vi "Controle_Manip_Main_GUI_WorkingBackup_211222.vi"() -> ()   [LabVIEW 2019] (continued)
                                }
                                frame #2 {
                                n1244 = local read "Spectrum End Wavelength (nm)"() -> (w1602:dbl)
                                n1245 = local read "Spectrum Step Wavelength (nm)"() -> (w1600:dbl)
                                n1246 = local read "Spectrum Start Wavelength (nm)"() -> (w1599:dbl)
                                n1247 = Subtract(x=w1602, y=w1599) -> (x-y=w1604:dbl)
                                n1248 = Divide(x=w1604, y=w1600) -> (x/y=w1603:dbl)
                                n1249 = Increment(x=w1603) -> (x+1=w1601:dbl)
                                n1250 = for {
                                N: w1601 -> [_]
                                tunnel: w1600 -> [w1607]
                                tunnel: w1599 -> [w1608]
                                shift-right: [w1609] -> w1595
                                shift-left: dbl[] [] -> [w1611]
                                shift-right: [w1612] -> w1596
                                shift-left: dbl[] [] -> [w1613]
                                i -> [w1617]
                                stop <- w1605 stop-if-true
                                n1251 = Multiply(x=w1617, y=w1607) -> (x*y=w1616:dbl)
                                n1252 = Add(x=w1608, y=w1616) -> (x+y=w1606:dbl)
                                n1253 = local read "ESP300 COM Port"() -> (w1615:refnum<visa-resource-name>)
                                n1254 = stacked-sequence {
                                tunnel: w1606 -> [w1620 _ w1627 _]
                                tunnel: w1615 -> [w1625 _ _ _]
                                tunnel: [_ _ w1634 _] -> w1614
                                tunnel: w1613 -> [w1623 _ _ _]
                                tunnel: [w1622 _ _ _] -> w1612
                                tunnel: [_ _ _ w1652] -> w1605
                                frame #0 {
                                w1618 = u16 1 items=["Detection"=1, "Excitation"=2] ("HR mode")
                                n1255 = call "MotorWL2Pos.vi"("Mono2 Center WL"=w1620, "HR mode"=w1618) -> ("Mono2 Position"=w1621:dbl)
                                n1256 = control-ref of="Mono2 Wavelength (nm)"() -> (w1619:refnum<vi>)
                                n1257 = control-ref of="Mono2 Motor Pos"() -> (w1624:refnum<vi>)
                                n1258 = call "subVI_Mono2Go2Posv2.vi"("Mono2 Motor Pos"=w1624, "Mono2 Wavelength (nm)"=w1619, "HR mode"=w1618, "Postion (Unit)"=w1621, "ESP300 COM Port"=w1625) -> ()  [unwired: 2 out]
                                n1259 = Insert Into Array(array=w1623, new element=w1620) -> (w1622:dbl[])  [unwired: 1 in]
                                }
                                frame #1 {
                                n1260 = Wait (ms)(milliseconds to wait=u32 20) -> ()  [unwired: 1 out]
                                }
                                frame #2 {
                                n1261 = local read "Photodiode error out"() -> (w1628:errorcluster)
                                n1262 = local read "Photodiode handle out"() -> (w1631:refnum<visa-resource-name>)
                                n1263 = Tick Count (ms)() -> (millisecond timer value=w1637:u32)
                                n1264 = call <instrlib>:"TLPM Set Wavelength.vi"("error in (no error)"=w1628, "Wavelength (0.0)"=w1627, "instrument handle"=w1631) -> ("error out"=w1629:errorcluster, "instrument handle out"=w1630:refnum<visa-resource-name>)  [unwired: 7 in]
                                n1265 = while {
                                shift-right: [w1647] -> w1632
                                shift-left: w1630 -> [w1650]
                                shift-right: [w1648] -> w1633
                                shift-left: w1629 -> [w1649]
                                tunnel: w1637 -> [w1645]
                                shift-right: [w1639] -> w1636
                                shift-left: dbl[] [] -> [w1640]
                                stop <- w1642 stop-if-true
                                n1266 = Tick Count (ms)() -> (millisecond timer value=w1646:u32)
                                n1267 = control-ref of="Excitation Power (uW)"() -> (w1638:refnum<vi>)
                                n1268 = local read "Acq Time (ms)"() -> (w1643:dbl)
                                n1269 = Subtract(x=w1646, y=w1645) -> (x-y=w1644:u32)
                                n1270 = call <instrlib>:"TLPM Measure Power.vi"("error in (no error)"=w1649, "instrument handle"=w1650) -> ("error out"=w1648:errorcluster, "Power"=w1641:dbl, "instrument handle out"=w1647:refnum<visa-resource-name>)  [unwired: 7 in]
                                n1271 = property class="DigNum (strict)"(reference=w1638, "Value"=w1641) -> ()  [unwired: 1 in, 2 out]
                                n1272 = Insert Into Array(array=w1640, new element=w1641) -> (w1639:dbl[])  [unwired: 1 in]
                                n1273 = Greater?(x=w1644, y=w1643) -> (0:w1642:bool)
                                }
                                n1274 = local write "Photodiode handle out"(w1632) -> ()
                                n1275 = local write "Photodiode error out"(w1633) -> ()
                                n1276 = call-poly <vilib>:"Mean.vi"("X"=w1636) -> ("mean"=w1634:dbl)  [unwired: 1 out]
                                }
                                frame #3 {
                                n1277 = control-ref of="MasterStop"() -> (w1651:refnum<vi>)
                                n1278 = control-ref of="Stop Spectrum Custom"() -> ()  [unwired: 1 out]
                                n1279 = property class="Bool (strict)"(reference=w1651) -> ("Value"=w1652:bool)  [unwired: 1 in, 2 out]
                                }
                                }
                                n1280 = Insert Into Array(array=w1611, new element=w1614) -> (w1609:dbl[])  [unwired: 1 in]
                                n1281 = Bundle(w1612, w1609) -> (w1610:cluster{dbl[], dbl[]})  [unwired: 1 in]
                                n1282 = property on="CCD 1D Spectrum Main" class="XYGraph (strict)"("Value"=w1610) -> ()  [unwired: 2 in, 2 out]
                                }
                                n1283 = local write "Data PL Custom Diode Spectrum"(w1595) -> ()
                                n1284 = local write "Wavelength calibration"(w1596) -> ()
                                }
                                frame #3 {
                                n1285 = property on="Elapsed (s)" class="DigNum (strict)"("Visible"=FALSE) -> ()  [unwired: 2 in, 2 out]
                                n1286 = control-ref of="Shutter Ctrls"() -> (w1655:refnum<vi>)
                                n1287 = local read "KCube Shutter On?"() -> (w1654:bool)
                                n1288 = control-ref of="KCube Shutter Device Reference"() -> (w1656:refnum<vi>)
                                n1289 = call "Shutter.vi"("KCube Shutter Device Reference 2"=w1656, "Shutter Ctrls 2"=w1655, "Shutter on?"=w1654) -> ()
                                }
                                }
                              }
                            }
                          }
                          frame #3 {
                            n1290 = property on="Save Custom Diode Spectrum" class="Bool (strict)"("Visible"=TRUE) -> ()  [unwired: 2 in, 2 out]
                            n1291 = control-ref of="MasterPause"() -> (w1658:refnum<vi>)
                            n1292 = control-ref of="MasterStop"() -> (w1660:refnum<vi>)
                            n1293 = local read "Scan Spectrum Cust Params"() -> (w1664:refnum<vi>[])
                            n1294 = property on="Acquire Custom Diode Spectrum" class="Bool (strict)"("Value"=FALSE ("Acquire Custom Diode Spectrum")) -> ()  [unwired: 2 in, 2 out]
                            n1295 = control-ref of="ExperimentStopped?"() -> (w1659:refnum<vi>)
                            n1296 = call "CheckStopAndReset.vi"("ExperimentStopped?"=w1659, "MasterStop"=w1660, "MasterPause"=w1658) -> ()
                            n1297 = call "Enable&Disable_Controls.vi"("Enum"=enum16{"Enabled", "Disabled", "Disabled&Grayed"}."Enabled", "References"=w1664) -> ()  [unwired: 1 in]
                            n1298 = local write "Background taken?"(FALSE ("Background taken?")) -> ()
                          }
                        }
                      }
                      frame "Acquire PLE" {
                        n1299 = stacked-sequence {
                          frame #0 {
                            # "background"
                            n1300 = local read "Background taken?"() -> (w1665:bool)
                            n1301 = case shown="False" w1665 {
                              frame False {
                                n1302 = stacked-sequence {
                                tunnel: [_ _ w1711] -> w1666
                                frame #0 {
                                n1303 = property on="CCD 1D Spectrum Main" class="XYGraph (strict)"("YScale.Offset"=0.0 ("Y Scale.Offset and Multiplier:Offset")) -> ()  [unwired: 2 in, 2 out]
                                }
                                frame #1 {
                                # "make sure shutter is closed"
                                n1304 = local read "KCube Shutter On?"() -> (w1697:bool)
                                n1305 = control-ref of="Shutter Ctrls"() -> (w1701:refnum<vi>)
                                n1306 = property class="Ring (strict)"(reference=w1701) -> ("Value"=w1700:u16)  [unwired: 1 in, 2 out]
                                n1307 = control-ref of="KCube Shutter Device Reference"() -> (w1702:refnum<vi>)
                                n1308 = Equal?(x=w1700, y=u16 0) -> (x = y?=w1698:bool)
                                n1309 = case shown="False" w1698 {
                                tunnel: w1702 -> [w1705 _]
                                tunnel: w1701 -> [w1704 _]
                                tunnel: w1697 -> [w1703 _]
                                frame False {
                                n1310 = call "Shutter.vi"("KCube Shutter Device Reference 2"=w1705, "Shutter Ctrls 2"=w1704, "Shutter on?"=w1703) -> ()
                                }
                                frame True {
                                }
                                }
                                }
                                frame #2 {
                                # "acquire"
                                n1311 = local read "LightField Automation error out"() -> (w1709:errorcluster)
                                n1312 = local read "LightField Automation out"() -> (w1710:refnum<class "LightField Automation.lvclass">)
                                n1313 = local read "Accumulations"() -> (w1706:dbl)
                                n1314 = call "LFA_Capture.vi"("error in (no error)"=w1709, "Frames"=w1706, "LightField Automation in"=w1710) -> ("error out"=w1708:errorcluster, "Data"=w1711:T26, "LightField Automation out"=w1707:refnum<class "LightField Automation.lvclass">)  [unwired: 6 in]
                                n1315 = local write "LightField Automation error out"(w1708) -> ()
                                n1316 = local write "LightField Automation out"(w1707) -> ()
                                }
                                }
                                n1317 = local read "Acq Mode"() -> (w1667:T3)
                                n1318 = case shown="\"Spectrum\", Default" w1667 {
                                selector: w1667 -> [w1668 w1686]
                                tunnel: w1666 -> [w1669 w1687]
                                frame "Spectrum", Default {
                                n1319 = stacked-sequence {
                                tunnel: w1669 -> [_ w1680 _ _]
                                tunnel: w1668 -> [_ w1678 _ _]
                                frame #0 {
                                n1320 = property on="CCD 2D Image Main" class="IntGraph (strict)"("Visible"=FALSE) -> ()  [unwired: 2 in, 2 out]
                                n1321 = property on="CCD 1D Spectrum Main" class="XYGraph (strict)"("Visible"=TRUE) -> ()  [unwired: 2 in, 2 out]
                                }
                                frame #1 {
                                n1322 = local read "Wavelength calibration"() -> (w1677:dbl[])
                                n1323 = local read "CCD ROI"() -> (w1673:T20)
                                n1324 = Divide(x=1239.842, y=w1677) -> (x/y=w1675:dbl[])
                                n1325 = call "PrepareData4Graph.vi"("Wavelength nm"=w1675, "DataLF"=w1680, "CCD ROI"=w1673, "AcqMode"=w1678, "Data type"=T30."Spectre") -> ("Spectrum"=w1679:cluster{"Array 2":dbl[], "Array":dbl[]}, "PLInt out"=w1672:dbl[])  [unwired: 2 in, 2 out]
                                n1326 = local write "CCD 1D Spectrum Main"(w1679) -> ()
                                n1327 = local write "BackgroundSpec"(w1672) -> ()
                                }
                                frame #2 {
                                n1328 = local read "BackgroundSpec"() -> (w1681:dbl[])
                                n1329 = call-poly <vilib>:"Mean.vi"("X"=w1681) -> ("mean"=w1683:dbl)  [unwired: 1 out]
                                n1330 = Negate(x=w1683) -> (-x=w1682:dbl)
                                n1331 = property on="CCD 1D Spectrum Main" class="XYGraph (strict)"("YScale.Offset"=w1682) -> ()  [unwired: 2 in, 2 out]
                                }
                                frame #3 {
                                n1332 = local write "Background taken?"(TRUE ("Background taken?")) -> ()
                                n1333 = property on="Background substract" class="Enum (strict)"("Value"=enum16{"None", "Shutter"}."None" ("Background substract")) -> ()  [unwired: 2 in, 2 out]
                                }
                                }
                                }
                                frame "Image" {
                                n1334 = stacked-sequence {
                                tunnel: w1687 -> [_ w1695]
                                tunnel: w1686 -> [_ w1693]
                                frame #0 {
                                n1335 = property on="CCD 1D Spectrum Main" class="XYGraph (strict)"("Visible"=FALSE) -> ()  [unwired: 2 in, 2 out]
                                n1336 = property on="CCD 2D Image Main" class="IntGraph (strict)"("Visible"=TRUE) -> ()  [unwired: 2 in, 2 out]
                                }
                                frame #1 {
                                n1337 = local read "Wavelength calibration"() -> (w1694:dbl[])
                                n1338 = local read "CCD ROI"() -> (w1690:T20)
                                n1339 = call "PrepareData4Graph.vi"("Wavelength nm"=w1694, "DataLF"=w1695, "CCD ROI"=w1690, "AcqMode"=w1693, "Data type"=T30."Spectre") -> ("Intensity Graph"=w1692:dbl[][])  [unwired: 2 in, 3 out]
                                n1340 = local write "CCD 2D Image Main"(w1692) -> ()
                                }
                                }
                                }
                                }
                              }
                              frame True {
                              }
                            }
                          }
                          frame #1 {
                            # "prep"
                            n1341 = control-ref of="MasterStop"() -> (w1731:refnum<vi>)
                            n1342 = control-ref of="MasterPause"() -> (w1728:refnum<vi>)
                            n1343 = local read "Spectrum Custom Mode"() -> (w1735:u16)
                            n1344 = local read "KCube Shutter On?"() -> (w1734:bool)
                            n1345 = local read "PLE Step (nm)"() -> (w1713:dbl)
                            n1346 = local read "PLE End (nm)"() -> (w1722:dbl)
                            n1347 = local read "Acq Time (ms)"() -> (w1733:dbl)
                            n1348 = local read "PLE Start (nm)"() -> (w1721:dbl)
                            n1349 = property class="Bool (strict)"(reference=w1731, "Visible"=TRUE) -> ()  [unwired: 1 in, 2 out]
                            n1350 = property class="Bool (strict)"(reference=w1728, "Visible"=TRUE) -> ()  [unwired: 1 in, 2 out]
                            n1351 = control-ref of="PLE # Pts"() -> (w1719:refnum<vi>)
                            n1352 = Bundle("Acq Time (ms)"=w1733, "PLE Start (nm)"=w1721, "PLE Step (nm)"=w1713, "PLE End (nm)"=w1722, "Spectrum Custom Mode"=w1735, "KCube Shutter On?"=w1734) -> (→"Scan PLE":T34)  [unwired: 1 in]
                            n1353 = Max & Min(x=w1721, y=w1722) -> (max(x,y)=w1717:dbl, min(x,y)=w1712:dbl)
                            n1354 = local read "Scan PLE AllParams"() -> (w1720:refnum<vi>[])
                            n1355 = property on="Experiment Graph Controls" class="TabCtl (strict)"("Value"=T25."PLE" ("Experiment Graph Controls")) -> ()  [unwired: 2 in, 2 out]
                            n1356 = Build Array (concatenate)(w1720, w1719) -> (w1718:refnum<vi>[])
                            n1357 = control-ref of="Elapsed (s)"() -> (w1726:refnum<vi>)
                            n1358 = call "Enable&Disable_Controls.vi"("Enum"=enum16{"Enabled", "Disabled", "Disabled&Grayed"}."Disabled&Grayed", "References"=w1718) -> ()  [unwired: 1 in]
                            n1359 = property class="DigNum (strict)"(reference=w1726, "Visible"=TRUE) -> ()  [unwired: 1 in, 2 out]
                            n1360 = Add(x=w1717, y=w1713) -> (x+y=w1714:dbl)
                            n1361 = Add(x=w1717, y=w1713) -> (x+y=w1716:dbl)
                            n1362 = property on="PLE Normalised Intensity" class="IntGraph (strict)"("XScale.Multiplier"=w1713, "XScale.Offset"=w1712, "YScale.Maximum"=1340.0 ("Y Scale.Range:Maximum"), "XScale.Minimum"=w1712, "XScale.Maximum"=w1716) -> ()  [unwired: 2 in, 2 out]
                            n1363 = property on="PLE Raw Intensity" class="IntGraph (strict)"("XScale.Multiplier"=w1713, "XScale.Offset"=w1712, "YScale.Maximum"=1340.0 ("Y Scale.Range:Maximum"), "XScale.Minimum"=w1712, "XScale.Maximum"=w1716) -> ()  [unwired: 2 in, 2 out]
                            n1364 = property on="PLE Laser Excitation Power" class="WFGraph (strict)"("XScale.Multiplier"=w1713, "XScale.Offset"=w1712, "XScale.Minimum"=w1712, "XScale.Maximum"=w1714) -> ()  [unwired: 2 in, 2 out]
                            n1365 = property on="PLE Integrated emission efficiency" class="WFGraph (strict)"("XScale.Multiplier"=w1713, "XScale.Offset"=w1712, "XScale.Minimum"=w1712, "XScale.Maximum"=w1714) -> ()  [unwired: 2 in, 2 out]
                          }
                          frame #2 {
                            n1366 = local read "Scan PLE"() -> (w1755:T1)
                            n1367 = Unbundle By Name(w1755) -> ("Acq Time (ms)"=w1748:dbl, "PLE start (nm)"=w1749:dbl, "PLE step (nm)"=w1750:dbl, "PLE end (nm)"=w1754:dbl)  [unwired: 2 out]
                            n1368 = Subtract(x=w1754, y=w1749) -> (x-y=w1753:dbl)
                            n1369 = Get Date/Time In Seconds() -> (seconds since 1Jan1904=w1744:timestamp)
                            n1370 = Divide(x=w1753, y=w1750) -> (x/y=w1752:dbl)
                            n1371 = Increment(x=w1752) -> (x+1=w1751:dbl)
                            n1372 = for {
                              N: w1751 -> [w1761]
                              tunnel: w1750 -> [w1777]
                              tunnel: w1749 -> [w1775]
                              tunnel: w1748 -> [w1773]
                              shift-right: [w1771] -> w1737
                              shift-left: dbl[] [] -> [w1772]
                              shift-right: [w1769] -> w1741
                              shift-left: i32[][] [] -> [w1770]
                              shift-right: [w1767] -> w1740
                              shift-left: dbl[][] [] -> [w1768]
                              tunnel: w1744 -> [w1763]
                              shift-right: [w1759] -> w1742
                              shift-left: dbl[] [] -> [w1760]
                              shift-right: [w1757] -> w1738
                              shift-left: dbl[] [] -> [w1758]
                              i -> [w1766]
                              stop <- w1778 stop-if-true
                              n1373 = Multiply(x=w1766, y=w1777) -> (x*y=w1776:dbl)
                              n1374 = Add(x=w1775, y=w1776) -> (x+y=w1774:dbl)
                              n1375 = Increment(x=w1766) -> (x+1=w1762:i32)
                              n1376 = Divide(x=w1762, y=w1761) -> (x/y=w1756:dbl)
                              n1377 = stacked-sequence {
                                tunnel: w1774 -> [_ w1792 _ _ w1804 _ _ _]
                                tunnel: w1773 -> [_ _ _ _ _ _ _ _]
                                tunnel: w1772 -> [_ _ _ _ w1801 _ _ _]
                                tunnel: [_ _ _ _ w1800 _ _ _] -> w1771
                                tunnel: w1770 -> [_ _ _ _ _ w1834 _ _]
                                tunnel: [_ _ _ _ _ w1833 _ _] -> w1769
                                tunnel: w1768 -> [_ _ _ _ _ w1832 _ _]
                                tunnel: [_ _ _ _ _ w1831 _ _] -> w1767
                                tunnel: w1763 -> [w1785 _ _ _ _ _ _ _]
                                tunnel: w1762 -> [w1784 _ _ _ _ _ _ _]
                                tunnel: w1761 -> [w1783 _ _ _ _ _ _ _]
                                tunnel: w1760 -> [_ _ _ _ _ w1830 _ _]
                                tunnel: [_ _ _ _ _ w1829 _ _] -> w1759
                                tunnel: w1758 -> [_ w1791 _ _ _ _ _ _]
                                tunnel: [_ w1790 _ _ _ _ _ _] -> w1757
                                tunnel: w1756 -> [_ _ w1797 _ _ _ _ _]
                                frame #0 {
                                # "prep"
                                n1378 = control-ref of="Expected (s)"() -> (w1781:refnum<vi>)
                                n1379 = call "Expectedtime.vi"("N"=w1783, "I"=w1784, "Reference time"=w1785) -> ("Expected time"=w1780:dbl, "Elapsed time"=w1782:dbl)
                                n1380 = property on="Elapsed (s)" class="DigNum (strict)"("Value"=w1782) -> ()  [unwired: 2 in, 2 out]
                                n1381 = property class="DigNum (strict)"(reference=w1781, "Value"=w1780) -> ()  [unwired: 1 in, 2 out]
                                }
                                frame #1 {
                                # "move filter to WL and get real wavelength"
                                n1382 = local read "LLTFDevice Interface"() -> (w1793:refnum<k7>)
                                n1383 = control-ref of="Laser on?"() -> (w1794:refnum<vi>)
                                n1384 = call "testmove.vi"("p_TargetWavelength"=w1792, "reference"=w1793) -> ("CurrentWavelength"=w1786:dbl, "CurrentAngle"=w1787:dbl, "Device reference out"=w1788:refnum<k7>, "Device moved"=w1789:bool)  [unwired: 4 in, 2 out]
                                n1385 = local write "CurrentAngle"(w1787) -> ()
                                n1386 = call "ExcWL2LaserrColor.vi"("Wavelength (380 - 780)"=w1792, "Laser on?"=w1794) -> ()  [unwired: 1 in]
                                n1387 = local write "CurrentWL"(w1786) -> ()
                                n1388 = local write "Device moved"(w1789) -> ()
                                n1389 = local write "LLTFDevice Interface"(w1788) -> ()
                                n1390 = Insert Into Array(array=w1791, new element=w1786) -> (w1790:dbl[])  [unwired: 1 in]
                                }
                                frame #2 {
                                # "move microscope objective to focus exc spot"
                                n1391 = local read "KCubePiezoDevice Z Reference"() -> (w1798:refnum<k24>)
                                n1392 = Multiply(x=w1797, y="FocalShift (V KCube)") -> (x*y=w1795:dbl)
                                n1393 = invoke class="KCubePiezo" method="SetOutputVoltage"(reference=w1798, "volts"=w1795) -> ()  [unwired: 2 in, 4 out]
                                }
                                frame #3 {
                                n1394 = Wait (ms)(milliseconds to wait=u32 50) -> ()  [unwired: 1 out]
                                }
                                frame #4 {
                                # "set excwl and measure power"
                                n1395 = local write "Excitation Wavelength (nm)"(w1804) -> ()
                                n1396 = local read "Photodiode Status"() -> (w1802:bool)
                                n1397 = case shown="True" w1802 {
                                tunnel: w1804 -> [_ w1811]
                                tunnel: w1801 -> [w1807 w1810]
                                tunnel: [w1805 w1809] -> w1800
                                frame False {
                                n1398 = Insert Into Array(array=w1807, new element=nan) -> (w1805:dbl[])  [unwired: 1 in]
                                }
                                frame True {
                                n1399 = local read "Photodiode handle out"() -> (w1817:refnum<visa-resource-name>)
                                n1400 = local read "Photodiode error out"() -> (w1816:errorcluster)
                                n1401 = call <instrlib>:"TLPM Set Wavelength.vi"("error in (no error)"=w1816, "Wavelength (0.0)"=w1811, "instrument handle"=w1817) -> ("error out"=w1815:errorcluster, "instrument handle out"=w1814:refnum<visa-resource-name>)  [unwired: 7 in]
                                n1402 = call <instrlib>:"TLPM Measure Power.vi"("error in (no error)"=w1815, "instrument handle"=w1814) -> ("error out"=w1812:errorcluster, "Power"=w1808:dbl, "instrument handle out"=w1813:refnum<visa-resource-name>)  [unwired: 7 in]
                                n1403 = local write "Photodiode handle out"(w1813) -> ()
                                n1404 = local write "Photodiode error out"(w1812) -> ()
                                n1405 = local write "Excitation Power (uW)"(w1808) -> ()
                                n1406 = Insert Into Array(array=w1810, new element=w1808) -> (w1809:dbl[])  [unwired: 1 in]
                                }
                                }
                                "PLE Laser Excitation Power" <- w1800
                                n1407 = control-ref of="Laser on?"() -> (w1803:refnum<vi>)
                                n1408 = call "ExcWL2LaserrColor.vi"("Wavelength (380 - 780)"=w1804, "Laser on?"=w1803) -> ()  [unwired: 1 in]
                                }
                                frame #5 {
                                # "acquire"
                                n1409 = stacked-sequence {
                                tunnel: [_ _ _ w1857] -> w1822
                                tunnel: [_ _ _ w1856] -> w1823
                                frame #0 {
                                # "open shutter if closed"
                                n1410 = control-ref of="KCube Shutter Device Reference"() -> (w1837:refnum<vi>)
                                n1411 = control-ref of="Shutter Ctrls"() -> (w1836:refnum<vi>)
                                n1412 = local read "KCube Shutter On?"() -> (w1835:bool)
                                n1413 = property class="Ring (strict)"(reference=w1836) -> ("Value"=w1838:u16)  [unwired: 1 in, 2 out]
                                n1414 = Equal?(x=w1838, y=u16 0) -> (x = y?=w1840:bool)
                                n1415 = case shown="True" w1840 {
                                tunnel: w1837 -> [_ w1843]
                                tunnel: w1836 -> [_ w1842]
                                tunnel: w1835 -> [_ w1841]
                                frame False {
                                }
                                frame True {
                                n1416 = call "Shutter.vi"("KCube Shutter Device Reference 2"=w1843, "Shutter Ctrls 2"=w1842, "Shutter on?"=w1841) -> ()
                                }
                                }
                                }
                                frame #1 {
                                # "set CCD ROI and acquire"
                                n1417 = local read "LightField Automation error out"() -> (w1852:errorcluster)
                                n1418 = local read "LightField Automation out"() -> (w1844:refnum<class "LightField Automation.lvclass">)
                                n1419 = local read "CCD ROI"() -> (w1851:T20)
                                n1420 = local read "Accumulations"() -> (w1848:dbl)
                                n1421 = call "Adv_SetROI.vi"("error in (no error)"=w1852, "ROI"=w1851, "LightField Automation in"=w1844) -> ("error out"=w1849:errorcluster, "LightField Automation out"=w1850:refnum<class "LightField Automation.lvclass">)  [unwired: 7 in]
                                n1422 = call "LFA_Capture.vi"("error in (no error)"=w1849, "Frames"=w1848, "LightField Automation in"=w1850) -> ("error out"=w1847:errorcluster, "Data"=w1846:T26, "LightField Automation out"=w1845:refnum<class "LightField Automation.lvclass">)  [unwired: 6 in]
                                n1423 = local write "LightField Automation error out"(w1847) -> ()
                                n1424 = local write "LightField Automation out"(w1845) -> ()
                                n1425 = local write "Data"(w1846) -> ()
                                }
                                frame #2 {
                                # "close shutter"
                                n1426 = local read "KCube Shutter On?"() -> (w1855:bool)
                                n1427 = control-ref of="KCube Shutter Device Reference"() -> (w1854:refnum<vi>)
                                n1428 = control-ref of="Shutter Ctrls"() -> (w1853:refnum<vi>)
                                n1429 = call "Shutter.vi"("KCube Shutter Device Reference 2"=w1854, "Shutter Ctrls 2"=w1853, "Shutter on?"=w1855) -> ()
                                }
                                frame #3 {
                                # "Show data accordingly"
                                n1430 = local read "Data"() -> (w1858:T26)
                                n1431 = local read "Acq Mode"() -> (w1859:T3)
                                n1432 = case shown="\"Spectrum\", Default" w1859 {
                                selector: w1859 -> [w1862 w1880]
                                tunnel: w1858 -> [w1863 w1881]
                                tunnel: [w1861 w1879] -> w1857
                                tunnel: [w1860 w1878] -> w1856
                                frame "Spectrum", Default {
                                n1433 = stacked-sequence {
                                tunnel: w1863 -> [_ w1877 _]
                                tunnel: w1862 -> [_ w1876 _]
                                tunnel: [_ w1866 _] -> w1861
                                tunnel: [_ w1865 _] -> w1860
                                frame #0 {
                                }
                                frame #1 {
                                w1864 = u16 4 items=["Sum", "Max", "Sum/s", "Max/s", "Efficiency"] ("Display Mode")
                                n1434 = local read "Excitation Power (uW)"() -> (w1868:dbl)
                                n1435 = local read "Wavelength calibration"() -> (w1875:dbl[])
                                n1436 = local read "CCD ROI"() -> (w1871:T20)
                                n1437 = local read "BackgroundSpec"() -> (w1867:dbl[])
                                n1438 = local read "Acq Time (ms)"() -> (w1869:dbl)
                                n1439 = Divide(x=1239.842, y=w1875) -> (x/y=w1873:dbl[])
                                n1440 = call "PrepareData4Graph.vi"("Wavelength nm"=w1873, "DataLF"=w1877, "CCD ROI"=w1871, "AcqMode"=w1876, "Data type"=T30."Spectre") -> ("PLInt out"=w1866:dbl[])  [unwired: 2 in, 3 out]
                                n1441 = control-ref of="Cnts"() -> (w1870:refnum<vi>)
                                n1442 = call "2Cnts.vi"("Array Background"=w1867, "Pow W"=w1868, "AcqTime ms"=w1869, "Cnts Ref"=w1870, "Display Mode"=w1864, "Array"=w1866) -> ("Value"=w1865:dbl)
                                }
                                frame #2 {
                                }
                                }
                                }
                                frame "Image" {
                                n1443 = stacked-sequence {
                                tunnel: w1881 -> [_ w1890]
                                tunnel: w1880 -> [_ w1888]
                                tunnel: [_ w1885] -> w1879
                                tunnel: [_ nan] -> w1878
                                frame #0 {
                                n1444 = property on="CCD 1D Spectrum Main" class="XYGraph (strict)"("Visible"=FALSE) -> ()  [unwired: 2 in, 2 out]
                                n1445 = property on="CCD 2D Image Main" class="IntGraph (strict)"("Visible"=TRUE) -> ()  [unwired: 2 in, 2 out]
                                }
                                frame #1 {
                                n1446 = local read "Wavelength calibration"() -> (w1889:dbl[])
                                n1447 = local read "CCD ROI"() -> (w1886:T20)
                                n1448 = call "PrepareData4Graph.vi"("Wavelength nm"=w1889, "DataLF"=w1890, "CCD ROI"=w1886, "AcqMode"=w1888, "Data type"=T30."Spectre") -> ("PLInt out"=w1885:dbl[])  [unwired: 2 in, 3 out]
                                }
                                }
                                }
                                }
                                }
                                }
                                n1449 = Insert Into Array(array=w1834, new element=w1822) -> (w1833:i32[][])  [unwired: 2 in]
                                "PLE Raw Intensity" <- w1833
                                n1450 = local read "BackgroundSpec"() -> (w1824:dbl[])
                                n1451 = local read "Excitation Power (uW)"() -> (w1820:dbl)
                                n1452 = local read "Acq Time (ms)"() -> (w1827:dbl)
                                n1453 = Multiply(x=w1820, y=1000000.0) -> (x*y=w1819:dbl)
                                n1454 = Divide(x=w1822, y=w1819) -> (x/y=w1818:dbl[])
                                n1455 = control-ref of="Cnts"() -> (w1828:refnum<vi>)
                                n1456 = Insert Into Array(array=w1832, new element=w1818) -> (w1831:dbl[][])  [unwired: 2 in]
                                "PLE Normalised Intensity" <- w1831
                                n1457 = control-ref of="Display Mode"() -> (w1826:refnum<vi>)
                                n1458 = property class="Ring (strict)"(reference=w1826) -> ("Value"=w1825:u16)  [unwired: 1 in, 2 out]
                                n1459 = call "2Cnts.vi"("Array Background"=w1824, "Pow W"=w1820, "AcqTime ms"=w1827, "Cnts Ref"=w1828, "Display Mode"=w1825, "Array"=w1822) -> ()  [unwired: 1 out]
                                n1460 = Insert Into Array(array=w1830, new element=w1823) -> (w1829:dbl[])  [unwired: 1 in]
                                "PLE Integrated emission efficiency" <- w1829
                                }
                                frame #6 {
                                # "datamanage"
                                }
                                frame #7 {
                                # "pause"
                                n1461 = while {
                                stop <- w1891 continue-if-true
                                n1462 = Wait (ms)(milliseconds to wait=u32 50) -> ()  [unwired: 1 out]
                                n1463 = local read "MasterPause"() -> (w1891:bool)
                                }
                                }
                              }
                              n1464 = Multiply(x=w1756, y=100.0) -> (x*y=w1764:dbl)
                              n1465 = property on="Scan Main Progess Bar" class="Slide (strict)"("Value"=w1764) -> ()  [unwired: 2 in, 2 out]
                              n1466 = control-ref of="MasterStop"() -> (w1779:refnum<vi>)
                              n1467 = property class="Bool (strict)"(reference=w1779) -> ("Value"=w1778:bool)  [unwired: 1 in, 2 out]
                            }
                            "PLE ExcPow" <- w1737
                            "PLE IntegInten" <- w1742
                            "PLE Raw Int" <- w1741
                            "PLE Norm Int" <- w1740
                            "PLE ExcWL" <- w1738
                            n1468 = Build Array(w1738, w1737) -> (→"PLE 2D ExcWL&Pow":dbl[][])
                          }
                          frame #3 {
                            n1469 = control-ref of="Save PLE"() -> (w1904:refnum<vi>)
                            n1470 = control-ref of="Acquire PLE"() -> (w1903:refnum<vi>)
                            n1471 = local read "Auto< ?"() -> (w1902:bool)
                            n1472 = case shown="False" w1902 {
                              tunnel: [TRUE ("Visible") FALSE ("Visible")] -> w1901
                              frame False {
                              }
                              frame True {
                              }
                            }
                            n1473 = control-ref of="MasterPause"() -> (w1905:refnum<vi>)
                            n1474 = control-ref of="MasterStop"() -> (w1907:refnum<vi>)
                            n1475 = property class="Bool (strict)"(reference=w1903, "Visible"=TRUE, "Value"=FALSE) -> ()  [unwired: 1 in, 2 out]
                            n1476 = property class="Bool (strict)"(reference=w1904, "Visible"=w1901) -> ()  [unwired: 1 in, 2 out]
                            n1477 = local read "Scan PLE AllParams"() -> (w1896:refnum<vi>[])
                            n1478 = control-ref of="ExperimentStopped?"() -> (w1906:refnum<vi>)
                            n1479 = call "CheckStopAndReset.vi"("ExperimentStopped?"=w1906, "MasterStop"=w1907, "MasterPause"=w1905) -> ()
                            n1480 = control-ref of="PLE # Pts"() -> (w1895:refnum<vi>)
                            n1481 = Build Array (concatenate)(w1896, w1895) -> (w1894:refnum<vi>[])
                            n1482 = control-ref of="Elapsed (s)"() -> (w1899:refnum<vi>)
                            n1483 = property class="DigNum (strict)"(reference=w1899, "Visible"=FALSE) -> ()  [unwired: 1 in, 2 out]
                            n1484 = call "Enable&Disable_Controls.vi"("Enum"=enum16{"Enabled", "Disabled", "Disabled&Grayed"}."Enabled", "References"=w1894) -> ()  [unwired: 1 in]
                          }
                        }
                      }
                      frame "Acquire Time Trace" {
                        n1485 = stacked-sequence {
                          frame #0 {
                            # "background"
                            n1486 = local read "Background taken?"() -> (w1910:bool)
                            n1487 = case shown="False" w1910 {
                              frame False {
                                n1488 = stacked-sequence {
                                tunnel: [_ _ w1960] -> w1911
                                frame #0 {
                                n1489 = local read "Log file"() -> (w1945:string)
                                n1490 = property on="CCD 1D Spectrum Main" class="XYGraph (strict)"("YScale.Offset"=0.0 ("Y Scale.Offset and Multiplier:Offset")) -> ()  [unwired: 2 in, 2 out]
                                n1491 = call "Write2LogFile.vi"("Add to log file"="Acquiring background", "Log file before"=w1945, "Checkbox"=FALSE) -> ("Log file after"=w1944:string)
                                n1492 = local write "Log file"(w1944) -> ()
                                }
                                frame #1 {
                                # "make sure shutter is closed"
                                n1493 = local read "KCube Shutter On?"() -> (w1946:bool)
                                n1494 = control-ref of="Shutter Ctrls"() -> (w1950:refnum<vi>)
                                n1495 = property class="Ring (strict)"(reference=w1950) -> ("Value"=w1949:u16)  [unwired: 1 in, 2 out]
                                n1496 = control-ref of="KCube Shutter Device Reference"() -> (w1951:refnum<vi>)
                                n1497 = Equal?(x=w1949, y=u16 0) -> (x = y?=w1947:bool)
                                n1498 = case shown="False" w1947 {
                                tunnel: w1951 -> [w1954 _]
                                tunnel: w1950 -> [w1953 _]
                                tunnel: w1946 -> [w1952 _]
                                frame False {
                                n1499 = call "Shutter.vi"("KCube Shutter Device Reference 2"=w1954, "Shutter Ctrls 2"=w1953, "Shutter on?"=w1952) -> ()
                                }
                                frame True {
                                }
                                }
                                }
                                frame #2 {
                                # "acquire"
                                n1500 = local read "LightField Automation error out"() -> (w1958:errorcluster)
                                n1501 = local read "LightField Automation out"() -> (w1959:refnum<class "LightField Automation.lvclass">)
                                n1502 = local read "Accumulations"() -> (w1955:dbl)
                                n1503 = call "LFA_Capture.vi"("error in (no error)"=w1958, "Frames"=w1955, "LightField Automation in"=w1959) -> ("error out"=w1957:errorcluster, "Data"=w1960:T26, "LightField Automation out"=w1956:refnum<class "LightField Automation.lvclass">)  [unwired: 6 in]
                                n1504 = local write "LightField Automation error out"(w1957) -> ()
                                n1505 = local write "LightField Automation out"(w1956) -> ()
                                }
                                }
                                n1506 = local read "Acq Mode"() -> (w1912:T3)
                                n1507 = case shown="\"Spectrum\", Default" w1912 {
                                selector: w1912 -> [w1913 w1931]
                                tunnel: w1911 -> [w1914 w1932]
                                frame "Spectrum", Default {
                                n1508 = stacked-sequence {
                                tunnel: w1914 -> [_ w1925 _ _]
                                tunnel: w1913 -> [_ w1923 _ _]
                                frame #0 {
                                n1509 = property on="CCD 2D Image Main" class="IntGraph (strict)"("Visible"=FALSE) -> ()  [unwired: 2 in, 2 out]
                                n1510 = property on="CCD 1D Spectrum Main" class="XYGraph (strict)"("Visible"=TRUE) -> ()  [unwired: 2 in, 2 out]
                                }
                                frame #1 {
                                n1511 = local read "Wavelength calibration"() -> (w1922:dbl[])
                                n1512 = local read "CCD ROI"() -> (w1918:T20)
                                n1513 = Divide(x=1239.842, y=w1922) -> (x/y=w1920:dbl[])
                                n1514 = call "PrepareData4Graph.vi"("Wavelength nm"=w1920, "DataLF"=w1925, "CCD ROI"=w1918, "AcqMode"=w1923, "Data type"=T30."Spectre") -> ("Spectrum"=w1924:cluster{"Array 2":dbl[], "Array":dbl[]}, "PLInt out"=w1917:dbl[])  [unwired: 2 in, 2 out]
                                n1515 = local write "CCD 1D Spectrum Main"(w1924) -> ()
                                n1516 = local write "BackgroundSpec"(w1917) -> ()
                                }
                                frame #2 {
                                n1517 = local read "BackgroundSpec"() -> (w1926:dbl[])
                                n1518 = call-poly <vilib>:"Mean.vi"("X"=w1926) -> ("mean"=w1928:dbl)  [unwired: 1 out]
                                n1519 = Negate(x=w1928) -> (-x=w1927:dbl)
                                n1520 = property on="CCD 1D Spectrum Main" class="XYGraph (strict)"("YScale.Offset"=w1927) -> ()  [unwired: 2 in, 2 out]
                                }
                                frame #3 {
                                n1521 = local write "Background taken?"(TRUE ("Background taken?")) -> ()
                                n1522 = property on="Background substract" class="Enum (strict)"("Value"=enum16{"None", "Shutter"}."None" ("Background substract")) -> ()  [unwired: 2 in, 2 out]
                                }
                                }
                                }
                                frame "Image" {
                                n1523 = stacked-sequence {
                                tunnel: w1932 -> [_ w1940]
                                tunnel: w1931 -> [_ w1938]
                                frame #0 {
                                n1524 = property on="CCD 1D Spectrum Main" class="XYGraph (strict)"("Visible"=FALSE) -> ()  [unwired: 2 in, 2 out]
                                n1525 = property on="CCD 2D Image Main" class="IntGraph (strict)"("Visible"=TRUE) -> ()  [unwired: 2 in, 2 out]
                                }
                                frame #1 {
                                n1526 = local read "Wavelength calibration"() -> (w1939:dbl[])
                                n1527 = local read "CCD ROI"() -> (w1935:T20)
                                n1528 = call "PrepareData4Graph.vi"("Wavelength nm"=w1939, "DataLF"=w1940, "CCD ROI"=w1935, "AcqMode"=w1938, "Data type"=T30."Spectre") -> ("Intensity Graph"=w1937:dbl[][])  [unwired: 2 in, 3 out]
                                n1529 = local write "CCD 2D Image Main"(w1937) -> ()
                                }
                                }
                                }
                                }
                              }
                              frame True {
                              }
                            }
                          }
                          frame #1 {
                            # "measurement"
                            n1530 = stacked-sequence {
                              frame #0 {
                                w1961 = FALSE ("Visible")
                                # "open shutter once"
                                n1531 = local read "KCube Shutter On?"() -> (w1962:bool)
                                n1532 = control-ref of="Shutter Ctrls"() -> (w1964:refnum<vi>)
                                n1533 = control-ref of="KCube Shutter Device Reference"() -> (w1963:refnum<vi>)
                                n1534 = call "Shutter.vi"("KCube Shutter Device Reference 2"=w1963, "Shutter Ctrls 2"=w1964, "Shutter on?"=w1962) -> ()
                                n1535 = property on="Acquire Time Trace" class="Bool (strict)"("Visible"=w1961) -> ()  [unwired: 2 in, 2 out]
                                n1536 = property on="Save Spectrum N" class="Bool (strict)"("Visible"=w1961) -> ()  [unwired: 2 in, 2 out]
                              }
                              frame #1 {
                                # "acquire N spectra"
                                n1537 = local read "CCD ROI"() -> (w1965:T20)
                                n1538 = local read "Acquire N: N"() -> (w1972:dbl)
                                n1539 = local read "LightField Automation error out"() -> (w1969:errorcluster)
                                n1540 = local read "LightField Automation out"() -> (w1968:refnum<class "LightField Automation.lvclass">)
                                n1541 = local read "Acq Mode"() -> (w1971:T3)
                                n1542 = call "LFA_Capture.vi"("error in (no error)"=w1969, "Frames"=w1972, "LightField Automation in"=w1968) -> ("error out"=w1966:errorcluster, "Data"=w1970:T26, "LightField Automation out"=w1967:refnum<class "LightField Automation.lvclass">)  [unwired: 6 in]
                                n1543 = case shown="\"Image\"" w1971 {
                                selector: w1971 -> [w1977 w1987]
                                tunnel: w1970 -> [w1979 w1988]
                                tunnel: w1965 -> [w1975 w1985]
                                frame "Spectrum", Default {
                                n1544 = local read "Wavelength calibration"() -> (w1978:dbl[])
                                n1545 = call "PrepareData4Graph.vi"("Wavelength nm"=w1978, "DataLF"=w1979, "CCD ROI"=w1975, "AcqMode"=w1977, "Data type"=T30."Time Trace") -> ("Intensity Graph"=w1974:dbl[][])  [unwired: 2 in, 3 out]
                                n1546 = Transpose 2D Array(2D array=w1974) -> (transposed array=w1973:dbl[][])
                                n1547 = local write "CCD 2D Image Main"(w1973) -> ()
                                }
                                frame "Image" {
                                n1548 = local read "Wavelength calibration"() -> (w1981:dbl[])
                                n1549 = Divide(x=1239.842, y=w1981) -> (x/y=w1980:dbl[])
                                n1550 = call "PrepareData4Graph.vi"("Wavelength nm"=w1980, "DataLF"=w1988, "CCD ROI"=w1985, "AcqMode"=w1987, "Data type"=T30."Time Trace") -> ("Intensity Graph"=w1984:dbl[][])  [unwired: 2 in, 3 out]
                                n1551 = Transpose 2D Array(2D array=w1984) -> (transposed array=w1983:dbl[][])
                                n1552 = local write "CCD 2D Image Main"(w1983) -> ()
                                }
                                }
                                n1553 = local write "LightField Automation error out"(w1966) -> ()
                                n1554 = local write "LightField Automation out"(w1967) -> ()
                                n1555 = local write "Data"(w1970) -> ()
                              }
                              frame #2 {
                                # "close shutter"
                                n1556 = local read "KCube Shutter On?"() -> (w1989:bool)
                                n1557 = control-ref of="Shutter Ctrls"() -> (w1991:refnum<vi>)
                                n1558 = control-ref of="KCube Shutter Device Reference"() -> (w1990:refnum<vi>)
                                n1559 = call "Shutter.vi"("KCube Shutter Device Reference 2"=w1990, "Shutter Ctrls 2"=w1991, "Shutter on?"=w1989) -> ()
                              }
                              frame #3 {
                                # "finish"
                                n1560 = property on="CCD 1D Spectrum Main" class="XYGraph (strict)"("Visible"=FALSE) -> ()  [unwired: 2 in, 2 out]
                                n1561 = property on="CCD 2D Image Main" class="IntGraph (strict)"("Visible"=TRUE) -> ()  [unwired: 2 in, 2 out]
                                n1562 = local read "Auto< ?"() -> (w1993:bool)
                                n1563 = Not(x=w1993) -> (.not. x?=w1994:bool)
                                n1564 = property on="Save Spectrum N" class="Bool (strict)"("Visible"=w1994) -> ()  [unwired: 2 in, 2 out]
                                n1565 = property on="Acquire Time Trace" class="Bool (strict)"("Visible"=TRUE) -> ()  [unwired: 2 in, 2 out]
                              }
                            }
                          }
                        }
                      }
                      frame "Acquire Polarisation" {
                        n1566 = stacked-sequence {
                          frame #0 {
                            # "background"
                            n1567 = local read "Background taken?"() -> (w1997:bool)
                            n1568 = case shown="False" w1997 {
                              frame False {
                                n1569 = stacked-sequence {
                                tunnel: [_ _ w2047] -> w1998
                                frame #0 {
                                n1570 = local read "Log file"() -> (w2032:string)
                                n1571 = property on="CCD 1D Spectrum Main" class="XYGraph (strict)"("YScale.Offset"=0.0 ("Y Scale.Offset and Multiplier:Offset")) -> ()  [unwired: 2 in, 2 out]
                                n1572 = call "Write2LogFile.vi"("Add to log file"="Acquiring background", "Log file before"=w2032, "Checkbox"=FALSE) -> ("Log file after"=w2031:string)
                                n1573 = local write "Log file"(w2031) -> ()
                                }
                                frame #1 {
                                # "make sure shutter is closed"
                                n1574 = local read "KCube Shutter On?"() -> (w2033:bool)
                                n1575 = control-ref of="Shutter Ctrls"() -> (w2037:refnum<vi>)
                                n1576 = property class="Ring (strict)"(reference=w2037) -> ("Value"=w2036:u16)  [unwired: 1 in, 2 out]
                                n1577 = control-ref of="KCube Shutter Device Reference"() -> (w2038:refnum<vi>)
                                n1578 = Equal?(x=w2036, y=u16 0) -> (x = y?=w2034:bool)
                                n1579 = case shown="False" w2034 {
                                tunnel: w2038 -> [w2041 _]
                                tunnel: w2037 -> [w2040 _]
                                tunnel: w2033 -> [w2039 _]
                                frame False {
                                n1580 = call "Shutter.vi"("KCube Shutter Device Reference 2"=w2041, "Shutter Ctrls 2"=w2040, "Shutter on?"=w2039) -> ()
                                }
                                frame True {
                                }
                                }
                                }
                                frame #2 {
                                # "acquire"
                                n1581 = local read "LightField Automation error out"() -> (w2045:errorcluster)
                                n1582 = local read "LightField Automation out"() -> (w2046:refnum<class "LightField Automation.lvclass">)
                                n1583 = local read "Accumulations"() -> (w2042:dbl)
                                n1584 = call "LFA_Capture.vi"("error in (no error)"=w2045, "Frames"=w2042, "LightField Automation in"=w2046) -> ("error out"=w2044:errorcluster, "Data"=w2047:T26, "LightField Automation out"=w2043:refnum<class "LightField Automation.lvclass">)  [unwired: 6 in]
                                n1585 = local write "LightField Automation error out"(w2044) -> ()
                                n1586 = local write "LightField Automation out"(w2043) -> ()
                                }
                                }
                                n1587 = local read "Acq Mode"() -> (w1999:T3)
                                n1588 = case shown="\"Spectrum\", Default" w1999 {
                                selector: w1999 -> [w2000 w2018]
                                tunnel: w1998 -> [w2001 w2019]
                                frame "Spectrum", Default {
                                n1589 = stacked-sequence {
                                tunnel: w2001 -> [_ w2012 _ _]
                                tunnel: w2000 -> [_ w2010 _ _]
                                frame #0 {
                                n1590 = property on="CCD 2D Image Main" class="IntGraph (strict)"("Visible"=FALSE) -> ()  [unwired: 2 in, 2 out]
                                n1591 = property on="CCD 1D Spectrum Main" class="XYGraph (strict)"("Visible"=TRUE) -> ()  [unwired: 2 in, 2 out]
                                }
                                frame #1 {
                                n1592 = local read "Wavelength calibration"() -> (w2009:dbl[])
                                n1593 = local read "CCD ROI"() -> (w2005:T20)
                                n1594 = Divide(x=1239.842, y=w2009) -> (x/y=w2007:dbl[])
                                n1595 = call "PrepareData4Graph.vi"("Wavelength nm"=w2007, "DataLF"=w2012, "CCD ROI"=w2005, "AcqMode"=w2010, "Data type"=T30."Spectre") -> ("Spectrum"=w2011:cluster{"Array 2":dbl[], "Array":dbl[]}, "PLInt out"=w2004:dbl[])  [unwired: 2 in, 2 out]
                                n1596 = local write "CCD 1D Spectrum Main"(w2011) -> ()
                                n1597 = local write "BackgroundSpec"(w2004) -> ()
                                }
                                frame #2 {
                                n1598 = local read "BackgroundSpec"() -> (w2013:dbl[])
                                n1599 = call-poly <vilib>:"Mean.vi"("X"=w2013) -> ("mean"=w2015:dbl)  [unwired: 1 out]
                                n1600 = Negate(x=w2015) -> (-x=w2014:dbl)
                                n1601 = property on="CCD 1D Spectrum Main" class="XYGraph (strict)"("YScale.Offset"=w2014) -> ()  [unwired: 2 in, 2 out]
                                }
                                frame #3 {
                                n1602 = local write "Background taken?"(TRUE ("Background taken?")) -> ()
                                n1603 = property on="Background substract" class="Enum (strict)"("Value"=enum16{"None", "Shutter"}."None" ("Background substract")) -> ()  [unwired: 2 in, 2 out]
                                }
                                }
                                }
                                frame "Image" {
                                n1604 = stacked-sequence {
                                tunnel: w2019 -> [_ w2027]
                                tunnel: w2018 -> [_ w2025]
                                frame #0 {
                                n1605 = property on="CCD 1D Spectrum Main" class="XYGraph (strict)"("Visible"=FALSE) -> ()  [unwired: 2 in, 2 out]
                                n1606 = property on="CCD 2D Image Main" class="IntGraph (strict)"("Visible"=TRUE) -> ()  [unwired: 2 in, 2 out]
                                }
                                frame #1 {
                                n1607 = local read "Wavelength calibration"() -> (w2026:dbl[])
                                n1608 = local read "CCD ROI"() -> (w2022:T20)
                                n1609 = call "PrepareData4Graph.vi"("Wavelength nm"=w2026, "DataLF"=w2027, "CCD ROI"=w2022, "AcqMode"=w2025, "Data type"=T30."Spectre") -> ("Intensity Graph"=w2024:dbl[][])  [unwired: 2 in, 3 out]